vi "Controle_Manip_Main_GUI_Backup2.vi"() -> ()   [LabVIEW 2019] (continued)
                n2776 = Divide(x=w3436, y=100.0) -> (x/y=w3434:dbl)
                n2777 = Divide(x=w3439, y=299792458.0) -> (x/y=w3437:dbl)
                n2778 = local write "Conv/Wavenumber (m-1)"(w3434) -> ()
                n2779 = local write "Conv/Time (s)"(w3437) -> ()
              }
              frame "Conv/Wavenumber (m-1)" {
              }
            }
          }
          event "CCD ROI": Value Change {
            n2780 = event-data() -> ()  [unwired: 1 in, 6 out]
            n2781 = local read "LightField On?"() -> (w3445:bool)
            n2782 = case shown="True" w3445 {
              frame False {
              }
              frame True {
                n2783 = stacked-sequence {
                  frame #0 {
                    n2784 = property on="CCD ROI" class="Enum (strict)"("DisabledEnum"=T28."Disabled and Grayed Out" ("Disabled")) -> ()  [unwired: 2 in, 2 out]
                  }
                  frame #1 {
                    n2785 = local read "LightField Automation error out"() -> (w3449:errorcluster)
                    n2786 = local read "LightField Automation out"() -> (w3451:refnum<class "LightField Automation.lvclass">)
                    n2787 = local read "CCD ROI"() -> (w3450:T20)
                    n2788 = call "Adv_SetROI.vi"("error in (no error)"=w3449, "ROI"=w3450, "LightField Automation in"=w3451) -> ("error out"=w3448:errorcluster, "LightField Automation out"=w3447:refnum<class "LightField Automation.lvclass">)  [unwired: 7 in]
                    n2789 = local write "LightField Automation out"(w3447) -> ()
                    n2790 = local write "LightField Automation error out"(w3448) -> ()
                  }
                  frame #2 {
                    n2791 = property on="CCD ROI" class="Enum (strict)"("DisabledEnum"=T28."Enabled" ("Disabled")) -> ()  [unwired: 2 in, 2 out]
                  }
                }
              }
            }
          }
          event "Cryostat": Value Change {
            n2792 = event-data() -> ("NewVal"=w3453:enum16{"Montana", "Oxford"})  [unwired: 1 in, 5 out]
            n2793 = case shown="\"Montana\"" w3453 {
              frame "Oxford" {
                w3454 = FALSE
                n2794 = property on="FSM Up" class="Bool (strict)"("Visible"=w3454) -> ()  [unwired: 2 in, 2 out]
                n2795 = property on="FSM Left" class="Bool (strict)"("Visible"=w3454) -> ()  [unwired: 2 in, 2 out]
                n2796 = property on="FSM Axis Step" class="DigNum (strict)"("Visible"=w3454) -> ()  [unwired: 2 in, 2 out]
                n2797 = property on="FSM Down" class="Bool (strict)"("Visible"=w3454) -> ()  [unwired: 2 in, 2 out]
                n2798 = property on="FSM Right" class="Bool (strict)"("Visible"=w3454) -> ()  [unwired: 2 in, 2 out]
              }
              frame "Montana" {
                w3455 = TRUE
                n2799 = property on="FSM Up" class="Bool (strict)"("Visible"=w3455) -> ()  [unwired: 2 in, 2 out]
                n2800 = property on="FSM Left" class="Bool (strict)"("Visible"=w3455) -> ()  [unwired: 2 in, 2 out]
                n2801 = property on="FSM Axis Step" class="DigNum (strict)"("Visible"=w3455) -> ()  [unwired: 2 in, 2 out]
                n2802 = property on="FSM Down" class="Bool (strict)"("Visible"=w3455) -> ()  [unwired: 2 in, 2 out]
                n2803 = property on="FSM Right" class="Bool (strict)"("Visible"=w3455) -> ()  [unwired: 2 in, 2 out]
              }
            }
          }
          event "Excitation Power (uW)": Mouse Down; "Excitation Wavelength (nm)", "Excitation Source": Value Change {
            n2804 = event-data() -> ("CtlRef"=w3459:refnum<vi>)  [unwired: 1 in, 3 out]
            n2805 = property class="Num"(reference=w3459) -> ("Label.Text"=w3458:string)  [unwired: 1 in, 2 out]
            n2806 = case shown="\"Excitation Source\"" w3458 {
              tunnel: [w3460 w3461 w3472 w3497] -> w3456
              frame "False", Default {
                n2807 = local read "Excitation Wavelength (nm)"() -> (w3460:dbl)
              }
              frame "Excitation Power (uW)" {
                n2808 = local read "PM16-120 On?"() -> (w3462:bool)
                n2809 = case shown="True" w3462 {
                  tunnel: [w3463 w3464] -> w3461
                  frame False {
                    n2810 = local read "Excitation Wavelength (nm)"() -> (w3463:dbl)
                  }
                  frame True {
                    n2811 = local read "Excitation Wavelength (nm)"() -> (w3464:dbl)
                    n2812 = local read "Photodiode handle out"() -> (w3471:refnum<visa-resource-name>)
                    n2813 = local read "Photodiode error out"() -> (w3470:errorcluster)
                    n2814 = call <instrlib>:"TLPM Set Wavelength.vi"("error in (no error)"=w3470, "Wavelength (0.0)"=w3464, "instrument handle"=w3471) -> ("error out"=w3469:errorcluster, "instrument handle out"=w3468:refnum<visa-resource-name>)  [unwired: 7 in]
                    n2815 = call <instrlib>:"TLPM Measure Power.vi"("error in (no error)"=w3469, "instrument handle"=w3468) -> ("error out"=w3465:errorcluster, "Power"=w3467:dbl, "instrument handle out"=w3466:refnum<visa-resource-name>)  [unwired: 7 in]
                    n2816 = local write "Photodiode handle out"(w3466) -> ()
                    n2817 = local write "Photodiode error out"(w3465) -> ()
                    n2818 = local write "Excitation Power (uW)"(w3467) -> ()
                  }
                }
              }
              frame "Excitation Wavelength (nm)" {
                n2819 = stacked-sequence {
                  tunnel: [_ w3484] -> w3472
                  frame #0 {
                    n2820 = local read "Excitation Source"() -> (w3476:enum16{"P", "CW", "SK"})
                    n2821 = local read "LLTF On?"() -> (w3477:bool)
                    n2822 = Equal?(x=w3476, y=enum16{"P", "CW", "SK"}."SK") -> (x = y?=w3474:bool)
                    n2823 = And(x=w3477, y=w3474) -> (x .and. y?=w3473:bool)
                    n2824 = case shown="True" w3473 {
                      frame False {
                      }
                      frame True {
                        n2825 = local read "Excitation Wavelength (nm)"() -> (w3483:dbl)
                        n2826 = local read "LLTFDevice Interface"() -> (w3482:refnum<k7>)
                        n2827 = call "testmove.vi"("p_TargetWavelength"=w3483, "reference"=w3482) -> ("CurrentWavelength"=w3480:dbl, "CurrentAngle"=w3481:dbl, "Device reference out"=w3479:refnum<k7>, "Device moved"=w3478:bool)  [unwired: 4 in, 2 out]
                        n2828 = local write "LLTFDevice Interface"(w3479) -> ()
                        n2829 = local write "Device moved"(w3478) -> ()
                        n2830 = local write "CurrentAngle"(w3481) -> ()
                        n2831 = local write "CurrentWL"(w3480) -> ()
                      }
                    }
                  }
                  frame #1 {
                    n2832 = local read "PM16-120 On?"() -> (w3485:bool)
                    n2833 = case shown="True" w3485 {
                      tunnel: [w3486 w3487] -> w3484
                      frame False {
                        n2834 = local read "Excitation Wavelength (nm)"() -> (w3486:dbl)
                      }
                      frame True {
                        n2835 = local read "Excitation Wavelength (nm)"() -> (w3487:dbl)
                        n2836 = local read "Photodiode handle out"() -> (w3494:refnum<visa-resource-name>)
                        n2837 = local read "Photodiode error out"() -> (w3493:errorcluster)
                        n2838 = call <instrlib>:"TLPM Set Wavelength.vi"("error in (no error)"=w3493, "Wavelength (0.0)"=w3487, "instrument handle"=w3494) -> ("error out"=w3492:errorcluster, "instrument handle out"=w3491:refnum<visa-resource-name>)  [unwired: 7 in]
                        n2839 = call <instrlib>:"TLPM Measure Power.vi"("error in (no error)"=w3492, "instrument handle"=w3491) -> ("error out"=w3488:errorcluster, "Power"=w3490:dbl, "instrument handle out"=w3489:refnum<visa-resource-name>)  [unwired: 7 in]
                        n2840 = local write "Photodiode handle out"(w3489) -> ()
                        n2841 = local write "Photodiode error out"(w3488) -> ()
                        n2842 = local write "Excitation Power (uW)"(w3490) -> ()
                      }
                    }
                  }
                }
              }
              frame "Excitation Source" {
                n2843 = local read "Excitation Source"() -> (w3496:enum16{"P", "CW", "SK"})
                n2844 = local read "PM16-120 On?"() -> (w3498:bool)
                n2845 = case shown="Default" w3496 {
                  tunnel: [TRUE ("Laser on?") w3501] -> w3495
                  frame Default {
                  }
                  frame "CW" {
                    n2846 = local read "Laser on? Control"() -> (w3501:bool)
                    n2847 = local write "Excitation Wavelength (nm)"(448.5 ("Excitation Wavelength (nm)")) -> ()
                  }
                }
                n2848 = case shown="True" w3498 {
                  tunnel: [w3502 w3503] -> w3497
                  frame False {
                    n2849 = local read "Excitation Wavelength (nm)"() -> (w3502:dbl)
                  }
                  frame True {
                    n2850 = local read "Excitation Wavelength (nm)"() -> (w3503:dbl)
                    n2851 = local read "Photodiode handle out"() -> (w3510:refnum<visa-resource-name>)
                    n2852 = local read "Photodiode error out"() -> (w3509:errorcluster)
                    n2853 = call <instrlib>:"TLPM Set Wavelength.vi"("error in (no error)"=w3509, "Wavelength (0.0)"=w3503, "instrument handle"=w3510) -> ("error out"=w3508:errorcluster, "instrument handle out"=w3507:refnum<visa-resource-name>)  [unwired: 7 in]
                    n2854 = call <instrlib>:"TLPM Measure Power.vi"("error in (no error)"=w3508, "instrument handle"=w3507) -> ("error out"=w3504:errorcluster, "Power"=w3506:dbl, "instrument handle out"=w3505:refnum<visa-resource-name>)  [unwired: 7 in]
                    n2855 = local write "Photodiode handle out"(w3505) -> ()
                    n2856 = local write "Photodiode error out"(w3504) -> ()
                    n2857 = local write "Excitation Power (uW)"(w3506) -> ()
                  }
                }
                n2858 = local write "Laser on?"(w3495) -> ()
              }
            }
            n2859 = control-ref of="Laser on?"() -> (w3457:refnum<vi>)
            n2860 = call "ExcWL2LaserrColor.vi"("Wavelength (380 - 780)"=w3456, "Laser on?"=w3457) -> ()  [unwired: 1 in]
          }
          event "Exit mirror": Value Change {
            n2861 = event-data() -> ("NewVal"=w3511:u16)  [unwired: 1 in, 5 out]
            n2862 = local read "LightField On?"() -> (w3512:bool)
            n2863 = case shown="True" w3512 {
              tunnel: w3511 -> [_ w3519]
              frame False {
              }
              frame True {
                n2864 = stacked-sequence {
                  tunnel: w3519 -> [_ w3525 _]
                  tunnel: [_ w3524 _] -> w3514
                  tunnel: [_ w3523 _] -> w3513
                  frame #0 {
                    n2865 = control-ref of="Exit mirror"() -> (w3522:refnum<vi>)
                    n2866 = Build Array(w3522) -> (w3521:refnum<vi>[])
                    n2867 = call "Enable&Disable_Controls.vi"("Enum"=enum16{"Enabled", "Disabled", "Disabled&Grayed"}."Disabled&Grayed", "References"=w3521) -> ()  [unwired: 1 in]
                  }
                  frame #1 {
                    n2868 = case shown="4, Default" w3525 {
                      tunnel: [enum16{"Enabled", "Disabled", "Disabled&Grayed"}."Disabled&Grayed" ("Enum") enum16{"Enabled", "Disabled", "Disabled&Grayed"}."Enabled" ("Enum")] -> w3524
                      tunnel: [AcqMode."APD 1" ("Acq Mode") w3539] -> w3523
                      frame 5 {
                      }
                      frame 4, Default {
                        n2869 = property on="Acq Mode" class="Enum (strict)"() -> ("Value"=w3538:T3)  [unwired: 2 in, 2 out]
                        n2870 = Not Equal?(x=w3538, y=AcqMode."Image" ("Acq Mode")) -> (x != y?=w3536:bool)
                        n2871 = case shown="True" w3536 {
                          tunnel: [AcqMode."Image" ("Acq Mode") AcqMode."Spectrum" ("Acq Mode")] -> w3539
                          frame False {
                          }
                          frame True {
                          }
                        }
                      }
                    }
                    n2872 = local read "LightField Automation error out"() -> (w3533:errorcluster)
                    n2873 = local read "LightField Automation out"() -> (w3532:refnum<class "LightField Automation.lvclass">)
                    n2874 = call "spec_GetOpticalExitPort.vi"("error in (no error)"=w3533, "LightField Automation in"=w3532) -> ("error out"=w3530:errorcluster, "Exit Port Location"=w3529:T33, "LightField Automation out"=w3531:refnum<class "LightField Automation.lvclass">)  [unwired: 7 in]
                    n2875 = Equal?(x=w3529, y=w3525) -> (x = y?=w3528:bool)
                    n2876 = case shown="False" w3528 {
                      tunnel: w3531 -> [w3553 w3555]
                      tunnel: w3530 -> [w3552 w3554]
                      tunnel: w3525 -> [w3551 _]
                      tunnel: [w3544 w3555] -> w3527
                      tunnel: [w3543 w3554] -> w3526
                      frame False {
                        n2877 = call "spec_SetOpticalExitPort.vi"("error in (no error)"=w3552, "Exit Port Location"=w3551, "LightField Automation in"=w3553) -> ("error out"=w3546:errorcluster, "LightField Automation out"=w3545:refnum<class "LightField Automation.lvclass">)  [unwired: 7 in]
                        n2878 = call "spec_GetCenterWavelength.vi"("error in (no error)"=w3546, "LightField Automation in"=w3545) -> ("error out"=w3549:errorcluster, "Center Wavelength"=w3547:dbl, "LightField Automation out"=w3548:refnum<class "LightField Automation.lvclass">)  [unwired: 7 in]
                        n2879 = local write "Center Wavelength (nm)"(w3547) -> ()
                        n2880 = call "spec_getCalibration.vi"("error in (no error)"=w3549, "LightField Automation in"=w3548) -> ("error out"=w3543:errorcluster, "ColumnCalibration"=w3550:dbl[], "LightField Automation out"=w3544:refnum<class "LightField Automation.lvclass">)  [unwired: 7 in]
                        n2881 = local write "Wavelength calibration"(w3550) -> ()
                      }
                      frame True {
                      }
                    }
                    n2882 = local write "LightField Automation error out"(w3526) -> ()
                    n2883 = local write "LightField Automation out"(w3527) -> ()
                  }
                  frame #2 {
                    n2884 = property on="Exit mirror" class="Ring (strict)"() -> ("RingText.Text"=w3560:string)  [unwired: 2 in, 2 out]
                    n2885 = local read "Log file"() -> (w3564:string)
                    n2886 = control-ref of="Exit mirror"() -> (w3559:refnum<vi>)
                    n2887 = Concatenate Strings("Exit mirror set to " ("Add to log file"), w3560) -> (w3561:string)
                    n2888 = call "Write2LogFile.vi"("Add to log file"=w3561, "Log file before"=w3564, "Checkbox"=FALSE) -> ("Log file after"=w3563:string)
                    n2889 = Build Array(w3559) -> (w3558:refnum<vi>[])
                    n2890 = call "Enable&Disable_Controls.vi"("Enum"=enum16{"Enabled", "Disabled", "Disabled&Grayed"}."Enabled", "References"=w3558) -> ()  [unwired: 1 in]
                    n2891 = local write "Log file"(w3563) -> ()
                  }
                }
                n2892 = control-ref of="Accumulations"() -> (w3516:refnum<vi>)
                n2893 = control-ref of="CCD ROI"() -> (w3517:refnum<vi>)
                n2894 = control-ref of="Exposure Time (ms)"() -> (w3518:refnum<vi>)
                n2895 = Build Array(w3516, w3517, w3518) -> (w3515:refnum<vi>[])
                n2896 = call "Enable&Disable_Controls.vi"("Enum"=w3514, "References"=w3515) -> ()  [unwired: 1 in]
                n2897 = property on="Acq Mode" class="Enum (strict)"("Value"=w3513) -> ()  [unwired: 2 in, 2 out]
              }
            }
          }
          event "Exposure Time (ms)", "Acquire N: N": Value Change {
            n2898 = event-data() -> ("CtlRef"=w3568:refnum<vi>, "NewVal"=w3565:dbl)  [unwired: 1 in, 4 out]
            n2899 = property class="DigNum (strict)"(reference=w3568) -> ("Label.Text"=w3567:string)  [unwired: 1 in, 2 out]
            n2900 = local read "LightField On?"() -> (w3566:bool)
            n2901 = case shown="\"Exposure Time (ms)\"" w3567 {
              tunnel: w3565 -> [w3570 w3572]
              tunnel: w3566 -> [_ w3573]
              frame "Acquire N: N", Default {
                n2902 = local read "Acq Time (ms)"() -> (w3569:dbl)
                n2903 = call "unnecessary_multiplication.vi"("N"=w3570, "AcqTime ms"=w3569) -> ("AcqTime Total (s)"=w3571:dbl)
                n2904 = local write "Duration"(w3571) -> ()
              }
              frame "Exposure Time (ms)" {
                n2905 = case shown="True" w3573 {
                  tunnel: w3572 -> [_ w3585]
                  frame False {
                  }
                  frame True {
                    n2906 = local read "LightField Automation error out"() -> (w3592:errorcluster)
                    n2907 = local read "LightField Automation out"() -> (w3591:refnum<class "LightField Automation.lvclass">)
                    n2908 = Divide(x=w3585, y=1000.0) -> (x/y=w3586:dbl)
                    n2909 = call "Exp_CCD_GetExposureTime.vi"("error in (no error)"=w3592, "LightField Automation in"=w3591) -> ("error out"=w3587:errorcluster, "Exposure Time (s)"=w3590:dbl, "LightField Automation out"=w3588:refnum<class "LightField Automation.lvclass">)  [unwired: 7 in]
                    n2910 = Equal?(x=w3590, y=w3586) -> (x = y?=w3589:bool)
                    n2911 = case shown="False" w3589 {
                      tunnel: w3588 -> [w3595 w3605]
                      tunnel: w3587 -> [w3594 w3604]
                      tunnel: w3586 -> [w3596 _]
                      tunnel: w3585 -> [_ _]
                      frame False {
                        n2912 = stacked-sequence {
                          tunnel: w3596 -> [_ w3600 _]
                          tunnel: w3595 -> [_ w3599 _]
                          tunnel: w3594 -> [_ w3598 _]
                          frame #0 {
                            n2913 = property on="Exposure Time (ms)" class="DigNum (strict)"("DisabledEnum"=T28."Disabled and Grayed Out" ("Disabled")) -> ()  [unwired: 2 in, 2 out]
                          }
                          frame #1 {
                            n2914 = call "Exp_CCD_SetExposureTime.vi"("error in (no error)"=w3598, "Exposure Time (s)"=w3600, "LightField Automation in"=w3599) -> ("error out"=w3601:errorcluster, "LightField Automation out"=w3602:refnum<class "LightField Automation.lvclass">)  [unwired: 7 in]
                            n2915 = local write "LightField Automation out"(w3602) -> ()
                            n2916 = local write "LightField Automation error out"(w3601) -> ()
                          }
                          frame #2 {
                            n2917 = property on="Exposure Time (ms)" class="DigNum (strict)"("DisabledEnum"=T28."Enabled" ("Disabled")) -> ()  [unwired: 2 in, 2 out]
                          }
                        }
                      }
                      frame True {
                        n2918 = local write "LightField Automation out"(w3605) -> ()
                        n2919 = local write "LightField Automation error out"(w3604) -> ()
                      }
                    }
                  }
                }
                n2920 = disable-structure shown="Disabled" {
                  disable-tunnel: w3572 -> [w3579 _]
                  frame Disabled {
                    n2921 = local read "Scan Y Num. Pts"() -> (w3581:dbl)
                    n2922 = local read "Scan X Num. Pts"() -> (w3582:dbl)
                    n2923 = Divide(x=w3579, y=1000.0) -> (x/y=w3577:dbl)
                    n2924 = Multiply(x=w3581, y=w3582) -> (x*y=w3583:dbl)
                    n2925 = Add(x=w3577, y=0.17) -> (x+y=w3576:dbl)
                    n2926 = Multiply(x=w3576, y=w3583) -> (x*y=w3584:dbl)
                    n2927 = local write "Expected (s)"(w3584) -> ()
                  }
                  frame Enabled {
                  }
                }
                n2928 = local write "Acq Time (ms)"(w3572) -> ()
                n2929 = local read "Acquire N: N"() -> (w3574:dbl)
                n2930 = call "unnecessary_multiplication.vi"("N"=w3574, "AcqTime ms"=w3572) -> ("AcqTime Total (s)"=w3575:dbl)
                n2931 = local write "Duration"(w3575) -> ()
              }
            }
          }
          event "FSM Home": Mouse Down {
            n2932 = event-data() -> ()  [unwired: 1 in, 6 out]
            n2933 = local read "FSM 300 On?"() -> (w3606:bool)
            n2934 = case shown="True" w3606 {
              frame False {
              }
              frame True {
                w3608 = 0.0 ("Target Value (V)")
                w3607 = 0.0 ("Target Value (V)")
                n2935 = local read "FSM Y Task"() -> (w3609:refnum<k21>)
                n2936 = local read "FSM X Task"() -> (w3610:refnum<k21>)
                n2937 = call "FSMGoTo.vi"("Target Value (V)"=w3607, "FSM Task"=w3610) -> ()  [unwired: 1 out]
                n2938 = call "FSMGoTo.vi"("Target Value (V)"=w3608, "FSM Task"=w3609) -> ()  [unwired: 1 out]
                n2939 = local write "Scan X Readout (V)"(w3607) -> ()
                n2940 = local write "Scan Y Readout (V)"(w3608) -> ()
                n2941 = property on="XY Intensity Map" class="IntGraph (strict)"("Cursor.Cursor X"=w3607) -> ()  [unwired: 2 in, 2 out]
                n2942 = property on="XY Intensity Map" class="IntGraph (strict)"("Cursor.Cursor Y"=w3608) -> ()  [unwired: 2 in, 2 out]
              }
            }
          }
          event "FSM Up", "FSM Down", "FSM Left", "FSM Right": Mouse Down {
            n2943 = event-data() -> ("CtlRef"=w3612:refnum<vi>)  [unwired: 1 in, 7 out]
            n2944 = local read "FSM 300 On?"() -> (w3611:bool)
            n2945 = case shown="True" w3611 {
              tunnel: w3612 -> [_ w3617]
              frame False {
              }
              frame True {
                n2946 = property class="Bool (strict)"(reference=w3617) -> ("Label.Text"=w3615:string)  [unwired: 1 in, 2 out]
                n2947 = local read "FSM Axis Step"() -> (w3616:dbl)
                n2948 = case shown="\"FSM Down\"" w3615 {
                  tunnel: [w3621 w3625 w3629 w3633] -> w3614
                  tunnel: w3616 -> [w3619 w3623 w3627 w3631]
                  tunnel: [w3618 w3622 w3626 w3630] -> w3613
                  frame "FSM Up", Default {
                    n2949 = local read "Scan Y Readout (V)"() -> (w3620:dbl)
                    n2950 = Add(x=w3620, y=w3619) -> (x+y=w3618:dbl)
                    n2951 = local write "Scan Y Readout (V)"(w3618) -> ()
                    n2952 = property on="XY Intensity Map" class="IntGraph (strict)"("Cursor.Cursor Y"=w3618) -> ()  [unwired: 2 in, 2 out]
                    n2953 = local read "FSM Y Task"() -> (w3621:refnum<k21>)
                  }
                  frame "FSM Down" {
                    n2954 = local read "Scan Y Readout (V)"() -> (w3624:dbl)
                    n2955 = Subtract(x=w3624, y=w3623) -> (x-y=w3622:dbl)
                    n2956 = local write "Scan Y Readout (V)"(w3622) -> ()
                    n2957 = local read "FSM Y Task"() -> (w3625:refnum<k21>)
                    n2958 = property on="XY Intensity Map" class="IntGraph (strict)"("Cursor.Cursor Y"=w3622) -> ()  [unwired: 2 in, 2 out]
                  }
                  frame "FSM Left" {
                    n2959 = local read "Scan X Readout (V)"() -> (w3628:dbl)
                    n2960 = Subtract(x=w3628, y=w3627) -> (x-y=w3626:dbl)
                    n2961 = local write "Scan X Readout (V)"(w3626) -> ()
                    n2962 = property on="XY Intensity Map" class="IntGraph (strict)"("Cursor.Cursor X"=w3626) -> ()  [unwired: 2 in, 2 out]
                    n2963 = local read "FSM X Task"() -> (w3629:refnum<k21>)
                  }
                  frame "FSM Right" {
                    n2964 = local read "Scan X Readout (V)"() -> (w3632:dbl)
                    n2965 = Add(x=w3632, y=w3631) -> (x+y=w3630:dbl)
                    n2966 = local write "Scan X Readout (V)"(w3630) -> ()
                    n2967 = property on="XY Intensity Map" class="IntGraph (strict)"("Cursor.Cursor X"=w3630) -> ()  [unwired: 2 in, 2 out]
                    n2968 = local read "FSM X Task"() -> (w3633:refnum<k21>)
                  }
                }
                n2969 = call "FSMGoTo.vi"("Target Value (V)"=w3613, "FSM Task"=w3614) -> ()  [unwired: 1 out]
              }
            }
          }
          event "FSM X Axis Pos", "FSM Y Axis Pos": Value Change {
            # "Move steering mirror"
            n2970 = event-data() -> ("CtlRef"=w3636:refnum<vi>, "NewVal"=w3635:dbl)  [unwired: 1 in, 4 out]
            n2971 = local read "FSM 300 On?"() -> (w3634:bool)
            n2972 = case shown="True" w3634 {
              tunnel: w3636 -> [_ w3640]
              tunnel: w3635 -> [_ w3637]
              frame False {
              }
              frame True {
                n2973 = property class="DigNum (strict)"(reference=w3640) -> ("Label.Text"=w3639:string)  [unwired: 1 in, 2 out]
                n2974 = case shown="\"FSM Y Axis Pos\"" w3639 {
                  tunnel: [w3642 w3644] -> w3638
                  tunnel: w3637 -> [w3641 w3643]
                  frame "FSM Y Axis Pos" {
                    n2975 = local write "Scan Y Readout (V)"(w3641) -> ()
                    n2976 = property on="XY Intensity Map" class="IntGraph (strict)"("Cursor.Cursor Y"=w3641) -> ()  [unwired: 2 in, 2 out]
                    n2977 = local read "FSM Y Task"() -> (w3642:refnum<k21>)
                  }
                  frame "FSM X Axis Pos", Default {
                    n2978 = local write "Scan X Readout (V)"(w3643) -> ()
                    n2979 = property on="XY Intensity Map" class="IntGraph (strict)"("Cursor.Cursor X"=w3643) -> ()  [unwired: 2 in, 2 out]
                    n2980 = local read "FSM X Task"() -> (w3644:refnum<k21>)
                  }
                }
                n2981 = call "FSMGoTo.vi"("Target Value (V)"=w3637, "FSM Task"=w3638) -> ()  [unwired: 1 out]
              }
            }
          }
          event "Add location": Mouse Down {
            (unwired) FALSE
            w3647 = "\r"
            n2982 = event-data() -> ()  [unwired: 1 in, 8 out]
            n2983 = local read "Map Marker X Pos"() -> (w3651:i8)
            n2984 = local read "Map Marker Y Pos"() -> (w3652:i8)
            n2985 = Format Into String(w3651) -> (resulting string=w3650:string)  [unwired: 3 in, 1 out]
            n2986 = Format Into String(w3652) -> (resulting string=w3648:string)  [unwired: 3 in, 1 out]
            n2987 = Concatenate Strings(w3647, "### Location ", w3650, "x" ("string"), w3648, w3647) -> (w3646:string)
            n2988 = call "Write2Markdown.vi"("String"=w3646) -> ()
            "ExportMapPosition?" <- FALSE ("ExportMapPosition?")
          }
          event "Full scale": Value Change {
            n2989 = event-data() -> ()  [unwired: 1 in, 6 out]
            n2990 = stacked-sequence {
              frame #0 {
                w3662 = 1239.842
                n2991 = property on="CCD 1D Spectrum Main" class="XYGraph (strict)"() -> ("Value"=w3657:cluster{dbl[], dbl[]})  [unwired: 2 in, 2 out]
                n2992 = Unbundle(w3657) -> (w3656:dbl[])  [unwired: 1 out]
                n2993 = property on="CCD 1D Spectrum Main" class="XYGraph (strict)"("XScale.ScaleFit"=u8 1 ("X Scale.Scale Fit"), "YScale.Minimum"=0.0 ("Y Scale.Range:Minimum")) -> ("XScale.Minimum"=w3654:dbl, "XScale.Maximum"=w3659:dbl)  [unwired: 2 in, 2 out]
                n2994 = call "myMax.vi"("Array"=w3656) -> ("myMax"=w3655:dbl)  [unwired: 1 in]
                n2995 = Divide(x=w3662, y=w3654) -> (x/y=w3660:dbl)
                n2996 = Divide(x=w3662, y=w3659) -> (x/y=w3661:dbl)
                n2997 = property on="CCD 1D Spectrum Main" class="XYGraph (strict)"("YScale.Maximum"=w3655) -> ()  [unwired: 2 in, 2 out]
                n2998 = property on="CCD 1D Spectrum Main Energy Scale" class="XYGraph (strict)"("XScale.Maximum"=w3660, "XScale.Minimum"=w3661) -> ()  [unwired: 2 in, 2 out]
              }
              frame #1 {
                n2999 = property on="Full scale" class="Bool (strict)"("Value"=FALSE ("Full scale")) -> ()  [unwired: 2 in, 2 out]
              }
            }
          }
          event "Grating": Value Change {
            n3000 = event-data() -> ("NewVal"=w3666:string)  [unwired: 1 in, 5 out]
            n3001 = local read "LightField On?"() -> (w3665:bool)
            n3002 = case shown="True" w3665 {
              tunnel: w3666 -> [_ w3673]
              frame False {
              }
              frame True {
                n3003 = local read "LightField Automation error out"() -> (w3672:errorcluster)
                n3004 = local read "LightField Automation out"() -> (w3670:refnum<class "LightField Automation.lvclass">)
                n3005 = call "spec_GetGratings.vi"("error in (no error)"=w3672, "LightField Automation in"=w3670) -> ("error out"=w3671:errorcluster, "Current Grating"=w3668:string, "LightField Automation out"=w3669:refnum<class "LightField Automation.lvclass">)  [unwired: 6 in, 1 out]
                n3006 = Equal?(x=w3673, y=w3668) -> (x = y?=w3667:bool)
                n3007 = case shown="False" w3667 {
                  tunnel: w3673 -> [w3679 _]
                  tunnel: w3671 -> [w3678 w3705]
                  tunnel: w3669 -> [w3677 w3706]
                  frame False {
                    n3008 = stacked-sequence {
                      seq-local: [_ w3689 _ _ _] -> [_ _ w3694 _ _]
                      seq-local: [_ w3688 _ _ _] -> [_ _ w3693 _ _]
                      seq-local: [_ w3687 _ _ _] -> [_ _ w3690 _ _]
                      seq-local: [_ _ w3692 _ _] -> [_ _ _ w3702 _]
                      seq-local: [_ _ w3691 _ _] -> [_ _ _ w3701 _]
                      seq-local: [_ _ w3690 _ _] -> [_ _ _ w3699 _]
                      tunnel: w3677 -> [_ w3689 _ _ _]
                      tunnel: w3678 -> [_ w3688 _ _ _]
                      tunnel: w3679 -> [_ w3687 _ _ _]
                      tunnel: [_ _ _ w3702 _] -> w3684
                      tunnel: [_ _ _ w3701 _] -> w3683
                      frame #0 {
                        n3009 = property on="Grating" class="CmbBox"("DisabledEnum"=T28."Disabled and Grayed Out" ("Disabled")) -> ()  [unwired: 2 in, 2 out]
                      }
                      frame #1 {
                      }
                      frame #2 {
                        n3010 = call "spec_SetGrating.vi"("error in (no error)"=w3693, "GratingSelected"=w3690, "LightField Automation in"=w3694) -> ("error out"=w3691:errorcluster, "LightField Automation out"=w3692:refnum<class "LightField Automation.lvclass">)  [unwired: 7 in]
                      }
                      frame #3 {
                        n3011 = local read "Log file"() -> (w3698:string)
                        n3012 = Concatenate Strings("Grating changed to " ("string"), w3699) -> (w3697:string)
                        n3013 = call "Write2LogFile.vi"("Add to log file"=w3697, "Log file before"=w3698, "Checkbox"=FALSE) -> ("Log file after"=w3696:string)
                        n3014 = local write "Log file"(w3696) -> ()
                      }
                      frame #4 {
                        n3015 = property on="Background substract" class="Enum (strict)"("Val(Sgnl)"=enum16{"None", "Shutter"}."Shutter" ("Value (Signaling)")) -> ()  [unwired: 2 in, 2 out]
                        n3016 = property on="Grating" class="CmbBox"("DisabledEnum"=T28."Enabled" ("Disabled")) -> ()  [unwired: 2 in, 2 out]
                      }
                    }
                    n3017 = call "spec_GetCenterWavelength.vi"("error in (no error)"=w3683, "LightField Automation in"=w3684) -> ("error out"=w3682:errorcluster, "Center Wavelength"=w3680:dbl, "LightField Automation out"=w3681:refnum<class "LightField Automation.lvclass">)  [unwired: 7 in]
                    n3018 = local write "Center Wavelength (nm)"(w3680) -> ()
                    n3019 = local write "Background taken?"(FALSE ("Background taken?")) -> ()
                    n3020 = call "spec_getCalibration.vi"("error in (no error)"=w3682, "LightField Automation in"=w3681) -> ("error out"=w3676:errorcluster, "ColumnCalibration"=w3685:dbl[], "LightField Automation out"=w3675:refnum<class "LightField Automation.lvclass">)  [unwired: 7 in]
                    n3021 = local write "LightField Automation out"(w3675) -> ()
                    n3022 = local write "LightField Automation error out"(w3676) -> ()
                    n3023 = local write "Wavelength calibration"(w3685) -> ()
                  }
                  frame True {
                    n3024 = local write "LightField Automation out"(w3706) -> ()
                    n3025 = local write "LightField Automation error out"(w3705) -> ()
                  }
                }
              }
            }
          }
          event "Mono2 On": Value Change {
            n3026 = event-data() -> ("NewVal"=w3708:bool)  [unwired: 1 in, 5 out]
            n3027 = local read "ESP 300 On?"() -> (w3707:bool)
            n3028 = case shown="True" w3707 {
              tunnel: w3708 -> [_ w3709]
              frame False {
              }
              frame True {
                n3029 = case shown="True" w3709 {
                  frame False {
                    n3030 = stacked-sequence {
                      frame #0 {
                        n3031 = local read "ESP300 COM Port"() -> (w3713:refnum<visa-resource-name>)
                        n3032 = local read "ESP300 Error"() -> (w3714:errorcluster)
                        n3033 = call "Motor Off.vi"("error in (no error)"=w3714, "Axis"=1, "VISA resource name in"=w3713) -> ("error out"=w3711:errorcluster, "VISA resource name out"=w3710:refnum<visa-resource-name>)  [unwired: 7 in]
                        n3034 = local write "ESP300 Error"(w3711) -> ()
                        n3035 = local write "ESP300 COM Port"(w3710) -> ()
                      }
                      frame #1 {
                        n3036 = local read "Log file"() -> (w3717:string)
                        n3037 = call "Write2LogFile.vi"("Add to log file"="Mono2 motor turned off", "Log file before"=w3717, "Checkbox"=FALSE) -> ("Log file after"=w3718:string)
                        n3038 = local write "Log file"(w3718) -> ()
                      }
                    }
                  }
                  frame True {
                    n3039 = stacked-sequence {
                      frame #0 {
                        n3040 = local read "ESP300 COM Port"() -> (w3722:refnum<visa-resource-name>)
                        n3041 = local read "ESP300 Error"() -> (w3723:errorcluster)
                        n3042 = call "Motor On.vi"("error in (no error)"=w3723, "Axis"=1, "VISA resource name in"=w3722) -> ("error out"=w3720:errorcluster, "VISA resource name out"=w3719:refnum<visa-resource-name>)  [unwired: 7 in]
                        n3043 = local write "ESP300 Error"(w3720) -> ()
                        n3044 = local write "ESP300 COM Port"(w3719) -> ()
                      }
                      frame #1 {
                        n3045 = local read "Log file"() -> (w3726:string)
                        n3046 = call "Write2LogFile.vi"("Add to log file"="Mono2 motor turned on", "Log file before"=w3726, "Checkbox"=FALSE) -> ("Log file after"=w3727:string)
                        n3047 = local write "Log file"(w3727) -> ()
                      }
                    }
                  }
                }
              }
            }
          }
          event "Motor LinT On?", "Motor RotStage Exc On?", "Motor RotStage Det On?", "LinTFine Motor On?": Mouse Down {
            n3048 = event-data() -> ("CtlRef"=w3730:refnum<vi>)  [unwired: 1 in, 7 out]
            n3049 = property class="Bool (strict)"(reference=w3730) -> ("Label.Text"=w3729:string, "Value"=w3728:bool)  [unwired: 1 in, 2 out]
            n3050 = case shown="\"LinTFine Motor On?\"" w3729 {
              tunnel: w3728 -> [w3732 _ w3740 w3748 w3756]
              frame "Motor RotStage Exc On?" {
                n3051 = local read "ESP 301 On?"() -> (w3731:bool)
                n3052 = case shown="True" w3731 {
                  tunnel: w3732 -> [_ w3733]
                  frame False {
                  }
                  frame True {
                    n3053 = local read "ESP 301 COM Port"() -> (w3738:refnum<visa-resource-name>)
                    n3054 = local read "ESP 301 Error"() -> (w3737:errorcluster)
                    n3055 = call "Enable Disable Motor.vi"("error in (no error)"=w3737, "Action (F - OFF)"=w3733, "Axis (1)"=2, "VISA resource name"=w3738) -> ("error out"=w3735:errorcluster, "VISA resource name out"=w3736:refnum<visa-resource-name>)  [unwired: 2 in]
                    n3056 = local write "ESP 301 COM Port"(w3736) -> ()
                    n3057 = local write "ESP 301 Error"(w3735) -> ()
                  }
                }
              }
              frame Default {
                # "default do nothing"
              }
              frame "LinTFine Motor On?" {
                n3058 = local read "PZC200 On?"() -> (w3739:bool)
                n3059 = case shown="True" w3739 {
                  tunnel: w3740 -> [_ w3743]
                  frame False {
                  }
                  frame True {
                    n3060 = case shown="False" w3743 {
                      tunnel: ["1MF" "1MO" ("Command")] -> w3742
                      frame False {
                      }
                      frame True {
                      }
                    }
                    n3061 = local read "PZC200 Instrument Channel"() -> (w3744:string)
                    n3062 = call "SendCommand.vi"("Command"=w3742, "Instrument Channel"=w3744) -> ("Instrument Channel out"=w3741:string)  [unwired: 8 in, 1 out]
                    n3063 = local write "PZC200 Instrument Channel"(w3741) -> ()
                  }
                }
              }
              frame "Motor LinT On?" {
                n3064 = local read "ESP 301 On?"() -> (w3747:bool)
                n3065 = case shown="True" w3747 {
                  tunnel: w3748 -> [_ w3751]
                  frame False {
                  }
                  frame True {
                    n3066 = local read "ESP 301 COM Port"() -> (w3754:refnum<visa-resource-name>)
                    n3067 = local read "ESP 301 Error"() -> (w3753:errorcluster)
                    n3068 = call "Enable Disable Motor.vi"("error in (no error)"=w3753, "Action (F - OFF)"=w3751, "Axis (1)"=1, "VISA resource name"=w3754) -> ("error out"=w3749:errorcluster, "VISA resource name out"=w3750:refnum<visa-resource-name>)  [unwired: 2 in]
                    n3069 = local write "ESP 301 COM Port"(w3750) -> ()
                    n3070 = local write "ESP 301 Error"(w3749) -> ()
                  }
                }
              }
              frame "Motor RotStage Det On?" {
                n3071 = local read "ESP 301 On?"() -> (w3755:bool)
                n3072 = case shown="True" w3755 {
                  tunnel: w3756 -> [_ w3757]
                  frame False {
                  }
                  frame True {
                    n3073 = local read "ESP 301 COM Port"() -> (w3762:refnum<visa-resource-name>)
                    n3074 = local read "ESP 301 Error"() -> (w3761:errorcluster)
                    n3075 = call "Enable Disable Motor.vi"("error in (no error)"=w3761, "Action (F - OFF)"=w3757, "Axis (1)"=3, "VISA resource name"=w3762) -> ("error out"=w3759:errorcluster, "VISA resource name out"=w3760:refnum<visa-resource-name>)  [unwired: 2 in]
                    n3076 = local write "ESP 301 COM Port"(w3760) -> ()
                    n3077 = local write "ESP 301 Error"(w3759) -> ()
                  }
                }
              }
            }
          }
          event "PZC Position Readout (usteps)", "RotStage Exc Angle Readout (°)", "RotStage Det Angle Readout (°)", "Newport Linear Translation Stage Position Readout (mm)": Mouse Down {
            n3078 = event-data() -> ("CtlRef"=w3765:refnum<vi>)  [unwired: 1 in, 7 out]
            n3079 = property class="DigNum (strict)"(reference=w3765) -> ("Label.Text"=w3764:string)  [unwired: 1 in, 2 out]
            n3080 = case shown="\"RotStage Det Angle Readout (°)\"" w3764 {
              tunnel: [0.0 ("Position (units)") w3767 w3778 w3789 w3796] -> w3763
              frame "False", Default {
              }
              frame "RotStage Exc Angle Readout (°)" {
                n3081 = local read "ESP 301 On?"() -> (w3768:bool)
                n3082 = case shown="True" w3768 {
                  tunnel: [0.0 ("Position (units)") w3775] -> w3767
                  frame False {
                  }
                  frame True {
                    w3770 = 3 ("Axis (1)")
                    n3083 = local read "ESP 301 COM Port"() -> (w3773:refnum<visa-resource-name>)
                    n3084 = local read "ESP 301 Error"() -> (w3774:errorcluster)
                    n3085 = call "Read absolute position.vi"("error in (no error)"=w3774, "Axis (1)"=w3770, "VISA resource name"=w3773) -> ("error out"=w3771:errorcluster, "VISA resource name out"=w3772:refnum<visa-resource-name>)  [unwired: 2 in, 1 out]
                    n3086 = call "Read absolute position.vi"("error in (no error)"=w3771, "Axis (1)"=w3770, "VISA resource name"=w3772) -> ("error out"=w3776:errorcluster, "Position (units)"=w3775:dbl, "VISA resource name out"=w3777:refnum<visa-resource-name>)  [unwired: 2 in]
                    n3087 = local write "ESP 301 COM Port"(w3777) -> ()
                    n3088 = local write "RotStage Exc Angle Readout (°)"(w3775) -> ()
                    n3089 = local write "ESP 301 Error"(w3776) -> ()
                  }
                }
              }
              frame "RotStage Det Angle Readout (°)" {
                n3090 = local read "ESP 301 On?"() -> (w3779:bool)
                n3091 = case shown="True" w3779 {
                  tunnel: [0.0 ("Position (units)") w3786] -> w3778
                  frame False {
                  }
                  frame True {
                    w3781 = 2 ("Axis (1)")
                    n3092 = local read "ESP 301 COM Port"() -> (w3782:refnum<visa-resource-name>)
                    n3093 = local read "ESP 301 Error"() -> (w3785:errorcluster)
                    n3094 = call "Read absolute position.vi"("error in (no error)"=w3785, "Axis (1)"=w3781, "VISA resource name"=w3782) -> ("error out"=w3784:errorcluster, "VISA resource name out"=w3783:refnum<visa-resource-name>)  [unwired: 2 in, 1 out]
                    n3095 = call "Read absolute position.vi"("error in (no error)"=w3784, "Axis (1)"=w3781, "VISA resource name"=w3783) -> ("error out"=w3788:errorcluster, "Position (units)"=w3786:dbl, "VISA resource name out"=w3787:refnum<visa-resource-name>)  [unwired: 2 in]
                    n3096 = local write "ESP 301 COM Port"(w3787) -> ()
                    n3097 = local write "RotStage Det Angle Readout (°)"(w3786) -> ()
                    n3098 = local write "ESP 301 Error"(w3788) -> ()
                  }
                }
              }
              frame "Newport Linear Translation Stage Position Readout (mm)" {
                n3099 = local read "ESP 301 On?"() -> (w3790:bool)
                n3100 = case shown="True" w3790 {
                  tunnel: [0.0 ("Position (units)") w3795] -> w3789
                  frame False {
                  }
                  frame True {
                    n3101 = local read "ESP 301 COM Port"() -> (w3793:refnum<visa-resource-name>)
                    n3102 = local read "ESP 301 Error"() -> (w3792:errorcluster)
                    n3103 = call "Read Actual Position.vi"("error in (no error)"=w3792, "Axis (1)"=1, "VISA resource name"=w3793) -> ("Position (units)"=w3795:dbl)  [unwired: 2 in, 2 out]
                    n3104 = local write "Newport Linear Translation Stage Position Readout (mm)"(w3795) -> ()
                  }
                }
              }
              frame "PZC Position Readout (usteps) " {
                n3105 = local read "PZC200 On?"() -> (w3797:bool)
                n3106 = case shown="True" w3797 {
                  tunnel: [0 ("Position") w3799] -> w3796
                  frame False {
                  }
                  frame True {
                    n3107 = local read "PZC200 Instrument Channel"() -> (w3802:string)
                    n3108 = call "PZCGetPos.vi"("Instrument Channel"=w3802) -> ("Instrument Channel Out"=w3800:string, "Position"=w3799:i32, "error out"=w3801:errorcluster)  [unwired: 1 in]
                    n3109 = local write "PZC Error"(w3801) -> ()
                    n3110 = local write "PZC Position Readout (usteps)"(w3799) -> ()
                    n3111 = local write "PZC200 Instrument Channel"(w3800) -> ()
                  }
                }
              }
            }
            "Position (units)" <- w3763
          }
          event "Reset origins": Value Change {
            n3112 = event-data() -> ("NewVal"=w3803:bool)  [unwired: 1 in, 5 out]
            n3113 = case shown="True" w3803 {
              frame False {
              }
              frame True {
                n3114 = disable-structure shown="Disabled" {
                  frame Disabled {
                    n3115 = local read "PZC Position Readout (usteps)"() -> ()  [unwired: 1 out]
                    n3116 = local read "Newport Linear Translation Stage Position Readout (mm)"() -> ()  [unwired: 1 out]
                  }
                  frame Enabled {
                  }
                }
              }
            }
          }
          event "RotStage Exc Angle (°)", "RotStage Det Angle (°)", "Newport Linear Translation Stage Position (mm)", "Newport PZA12 Stage Position (usteps)": Value Change {
            n3117 = event-data() -> ("CtlRef"=w3806:refnum<vi>, "NewVal"=w3805:dbl)  [unwired: 1 in, 4 out]
            n3118 = property class="DigNum (strict)"(reference=w3806) -> ("Label.Text"=w3804:string)  [unwired: 1 in, 2 out]
            n3119 = case shown="\"RotStage Exc Angle (°)\"" w3804 {
              tunnel: w3804 -> [_ _ w3825 _ w3865 w3894]
              tunnel: w3805 -> [_ w3808 w3824 w3860 w3864 w3893]
              frame "False", Default {
              }
              frame "Newport PZA12 Stage Position (usteps)" {
                n3120 = local read "PZC200 On?"() -> (w3807:bool)
                n3121 = case shown="True" w3807 {
                  tunnel: w3808 -> [_ w3810]
                  frame False {
                  }
                  frame True {
                    n3122 = local read "PZC200 Instrument Channel"() -> (w3814:string)
                    n3123 = call "PZCGetPos.vi"("Instrument Channel"=w3814) -> ("Instrument Channel Out"=w3811:string, "Position"=w3813:i32)  [unwired: 1 in, 1 out]
                    n3124 = Not Equal?(x=w3810, y=w3813) -> (x != y?=w3812:bool)
                    n3125 = case shown="True" w3812 {
                      tunnel: w3811 -> [w3815 w3818]
                      tunnel: w3810 -> [_ w3817]
                      tunnel: [w3815 w3816] -> w3809
                      frame False {
                      }
                      frame True {
                        n3126 = stacked-sequence {
                          tunnel: w3818 -> [w3822]
                          tunnel: w3817 -> [w3821]
                          tunnel: [w3819] -> w3816
                          frame #0 {
                            n3127 = call "PZC_MoveAbs.vi"("Target"=w3821, "Instrument"=w3822) -> ("Final Position"=w3820:i32, "Instrument out"=w3819:string)  [unwired: 1 in, 1 out]
                            n3128 = local write "PZC Position Readout (usteps)"(w3820) -> ()
                          }
                        }
                      }
                    }
                    n3129 = local write "PZC200 Instrument Channel"(w3809) -> ()
                  }
                }
              }
              frame "Newport Linear Translation Stage Position (mm)" {
                n3130 = local read "ESP 301 On?"() -> (w3823:bool)
                n3131 = case shown="True" w3823 {
                  tunnel: w3825 -> [_ w3840]
                  tunnel: w3824 -> [_ w3829]
                  frame False {
                  }
                  frame True {
                    n3132 = case shown="\"Newport Linear Translation Stage Position (mm)\"" w3840 {
                      tunnel: [2 1 3] -> w3841
                      tunnel: [w3844 w3847 w3850] -> w3838
                      tunnel: w3829 -> [w3843 w3846 w3849]
                      frame "RotStage Det Angle (°)" {
                        n3133 = local write "RotStage Det Angle (°)"(w3843) -> ()
                        n3134 = control-ref of="RotStage Det Angle Readout (°)"() -> (w3844:refnum<vi>)
                      }
                      frame "Newport Linear Translation Stage Position (mm)" {
                        n3135 = control-ref of="Newport Linear Translation Stage Position Readout (mm)"() -> (w3847:refnum<vi>)
                        n3136 = local write "Newport Linear Translation Stage Position (mm)"(w3846) -> ()
                      }
                      frame "RotStage Exc Angle (°)", Default {
                        n3137 = local write "RotStage Exc Angle (°)"(w3849) -> ()
                        n3138 = control-ref of="RotStage Exc Angle Readout (°)"() -> (w3850:refnum<vi>)
                      }
                    }
                    n3139 = local read "Excitation Wavelength (nm)"() -> (w3834:dbl)
                    n3140 = local read "Photodiode Status"() -> (w3826:bool)
                    n3141 = local read "Photodiode handle out"() -> (w3836:refnum<visa-resource-name>)
                    n3142 = local read "Photodiode error out"() -> (w3835:errorcluster)
                    n3143 = local read "ESP 301 Error"() -> (w3842:errorcluster)
                    n3144 = control-ref of="Excitation Power (uW)"() -> (w3837:refnum<vi>)
                    n3145 = call <instrlib>:"TLPM Set Wavelength.vi"("error in (no error)"=w3835, "Wavelength (0.0)"=w3834, "instrument handle"=w3836) -> ("error out"=w3832:errorcluster, "instrument handle out"=w3833:refnum<visa-resource-name>)  [unwired: 7 in]
                    n3146 = local read "ESP 301 COM Port"() -> (w3828:refnum<visa-resource-name>)
                    n3147 = call "Go2Angle.vi"("VISA resource name"=w3828, "Photodiode"=w3833, "RotStage Det Angle Readout (°) 4"=w3838, "Excitation Power (uW) 2"=w3837, "Photodiode on?"=w3826, "Axis ESP301 / RotStage"=w3841, "ESP301 Error"=w3842, "Photodiode error"=w3832, "Position (units)"=w3829) -> ("Photodiode out"=w3830:refnum<visa-resource-name>, "VISA resource name out"=w3827:refnum<visa-resource-name>, "Photodiode"=w3831:errorcluster, "ESP301 Error out"=w3839:errorcluster)  [unwired: 3 in]
                    n3148 = local write "ESP 301 Error"(w3839) -> ()
                    n3149 = local write "Photodiode handle out"(w3830) -> ()
                    n3150 = local write "Photodiode error out"(w3831) -> ()
                    n3151 = local write "ESP 301 COM Port"(w3827) -> ()
                  }
                }
              }
              frame "Newport Linear Translation Stage Position (mm) Test" {
                w3855 = 1 ("Axis (1)")
                n3152 = local read "ESP 301 COM Port"() -> (w3859:refnum<visa-resource-name>)
                n3153 = local read "ESP 301 Error"() -> (w3858:errorcluster)
                n3154 = call "Move Absolute.vi"("error in (no error)"=w3858, "Position (0 units)"=w3860, "Axis (1)"=w3855, "VISA resource name"=w3859) -> ("error out"=w3861:errorcluster, "VISA resource name out"=w3862:refnum<visa-resource-name>)  [unwired: 2 in]
                n3155 = call "Wait For Motion Stop.vi"("error in (no error)"=w3861, "Axis (0)"=w3855, "VISA resource name"=w3862) -> ("error out"=w3856:errorcluster, "VISA resource name out"=w3857:refnum<visa-resource-name>)  [unwired: 3 in]
                n3156 = call "Read absolute position.vi"("error in (no error)"=w3856, "Axis (1)"=w3855, "VISA resource name"=w3857) -> ("error out"=w3853:errorcluster, "Position (units)"=w3852:dbl, "VISA resource name out"=w3854:refnum<visa-resource-name>)  [unwired: 2 in]
                n3157 = local write "Newport Linear Translation Stage Position Readout (mm)"(w3852) -> ()
                n3158 = local write "ESP 301 COM Port"(w3854) -> ()
                n3159 = local write "ESP 301 Error"(w3853) -> ()
              }
              frame "RotStage Exc Angle (°)" {
                n3160 = local read "ESP 301 On?"() -> (w3863:bool)
                n3161 = case shown="True" w3863 {
                  tunnel: w3865 -> [_ w3882]
                  tunnel: w3864 -> [_ w3881]
                  frame False {
                  }
                  frame True {
                    n3162 = case shown="\"RotStage Exc Angle (°)\", Default" w3882 {
                      tunnel: [2 1 3] -> w3878
                      tunnel: [w3884 w3887 w3890] -> w3875
                      tunnel: w3881 -> [w3883 w3886 w3889]
                      frame "RotStage Det Angle (°)" {
                        n3163 = local write "RotStage Det Angle (°)"(w3883) -> ()
                        n3164 = control-ref of="RotStage Det Angle Readout (°)"() -> (w3884:refnum<vi>)
                      }
                      frame "Newport Linear Translation Stage Position (mm)" {
                        n3165 = control-ref of="Newport Linear Translation Stage Position Readout (mm)"() -> (w3887:refnum<vi>)
                        n3166 = local write "Newport Linear Translation Stage Position (mm)"(w3886) -> ()
                      }
                      frame "RotStage Exc Angle (°)", Default {
                        n3167 = local write "RotStage Exc Angle (°)"(w3889) -> ()
                        n3168 = control-ref of="RotStage Exc Angle Readout (°)"() -> (w3890:refnum<vi>)
                      }
                    }
                    n3169 = local read "Excitation Wavelength (nm)"() -> (w3871:dbl)
                    n3170 = local read "Photodiode handle out"() -> (w3873:refnum<visa-resource-name>)
                    n3171 = local read "Photodiode error out"() -> (w3872:errorcluster)
                    n3172 = local read "Photodiode Status"() -> (w3866:bool)
                    n3173 = local read "ESP 301 Error"() -> (w3879:errorcluster)
                    n3174 = control-ref of="Excitation Power (uW)"() -> (w3874:refnum<vi>)
                    n3175 = call <instrlib>:"TLPM Set Wavelength.vi"("error in (no error)"=w3872, "Wavelength (0.0)"=w3871, "instrument handle"=w3873) -> ("error out"=w3869:errorcluster, "instrument handle out"=w3870:refnum<visa-resource-name>)  [unwired: 7 in]
                    n3176 = local read "ESP 301 COM Port"() -> (w3880:refnum<visa-resource-name>)
                    n3177 = call "Go2Angle.vi"("VISA resource name"=w3880, "Photodiode"=w3870, "RotStage Det Angle Readout (°) 4"=w3875, "Excitation Power (uW) 2"=w3874, "Photodiode on?"=w3866, "Axis ESP301 / RotStage"=w3878, "ESP301 Error"=w3879, "Photodiode error"=w3869, "Position (units)"=w3881) -> ("Photodiode out"=w3867:refnum<visa-resource-name>, "VISA resource name out"=w3877:refnum<visa-resource-name>, "Photodiode"=w3868:errorcluster, "ESP301 Error out"=w3876:errorcluster)  [unwired: 3 in]
                    n3178 = local write "Photodiode error out"(w3868) -> ()
                    n3179 = local write "ESP 301 Error"(w3876) -> ()
                    n3180 = local write "ESP 301 COM Port"(w3877) -> ()
                    n3181 = local write "Photodiode handle out"(w3867) -> ()
                  }
                }
              }
              frame "RotStage Det Angle (°)" {
                n3182 = local read "ESP 301 On?"() -> (w3892:bool)
                n3183 = case shown="True" w3892 {
                  tunnel: w3894 -> [_ w3908]
                  tunnel: w3893 -> [_ w3896]
                  frame False {
                  }
                  frame True {
                    n3184 = case shown="\"RotStage Exc Angle (°)\", Default" w3908 {
                      tunnel: [2 1 3] -> w3909
                      tunnel: [w3913 w3916 w3919] -> w3905
                      tunnel: w3896 -> [w3912 w3915 w3918]
                      frame "RotStage Det Angle (°)" {
                        n3185 = local write "RotStage Det Angle (°)"(w3912) -> ()
                        n3186 = control-ref of="RotStage Det Angle Readout (°)"() -> (w3913:refnum<vi>)
                      }
                      frame "Newport Linear Translation Stage Position (mm)" {
                        n3187 = control-ref of="Newport Linear Translation Stage Position Readout (mm)"() -> (w3916:refnum<vi>)
                        n3188 = local write "Newport Linear Translation Stage Position (mm)"(w3915) -> ()
                      }
                      frame "RotStage Exc Angle (°)", Default {
                        n3189 = local write "RotStage Exc Angle (°)"(w3918) -> ()
                        n3190 = control-ref of="RotStage Exc Angle Readout (°)"() -> (w3919:refnum<vi>)
                      }
                    }
                    n3191 = local read "Excitation Wavelength (nm)"() -> (w3901:dbl)
                    n3192 = local read "Photodiode handle out"() -> (w3903:refnum<visa-resource-name>)
                    n3193 = local read "Photodiode error out"() -> (w3902:errorcluster)
                    n3194 = local read "Photodiode Status"() -> (w3895:bool)
                    n3195 = local read "ESP 301 Error"() -> (w3910:errorcluster)
                    n3196 = control-ref of="Excitation Power (uW)"() -> (w3904:refnum<vi>)
                    n3197 = call <instrlib>:"TLPM Set Wavelength.vi"("error in (no error)"=w3902, "Wavelength (0.0)"=w3901, "instrument handle"=w3903) -> ("error out"=w3899:errorcluster, "instrument handle out"=w3900:refnum<visa-resource-name>)  [unwired: 7 in]
                    n3198 = local read "ESP 301 COM Port"() -> (w3911:refnum<visa-resource-name>)
                    n3199 = call "Go2Angle.vi"("VISA resource name"=w3911, "Photodiode"=w3900, "RotStage Det Angle Readout (°) 4"=w3905, "Excitation Power (uW) 2"=w3904, "Photodiode on?"=w3895, "Axis ESP301 / RotStage"=w3909, "ESP301 Error"=w3910, "Photodiode error"=w3899, "Position (units)"=w3896) -> ("Photodiode out"=w3897:refnum<visa-resource-name>, "VISA resource name out"=w3907:refnum<visa-resource-name>, "Photodiode"=w3898:errorcluster, "ESP301 Error out"=w3906:errorcluster)  [unwired: 3 in]
                    n3200 = local write "ESP 301 COM Port"(w3907) -> ()
                    n3201 = local write "ESP 301 Error"(w3906) -> ()
                    n3202 = local write "Photodiode handle out"(w3897) -> ()